vi "UHR-Fleezers Control (host) - 12.0.vi"() -> ()   [LabVIEW 2014] (continued)
                                frame #2 {
                                n432 = property on="Load parameters" class="Bool (strict)"("Val(Sgnl)"=TRUE ("Value (Signaling)")) -> ()  [unwired: 2 in, 2 out]
                                n433 = case shown="True" "Green ON during\nraster?" {
                                frame False {
                                }
                                frame True {
                                n434 = property on="Green ON/Interlacing" class="Bool (strict)"("Val(Sgnl)"=TRUE ("Value (Signaling)")) -> ()  [unwired: 2 in, 2 out]
                                }
                                }
                                }
                                frame #3 {
                                n435 = Wait (ms)(milliseconds to wait=u32 500) -> ()  [unwired: 1 out]
                                }
                                frame #4 {
                                n436 = property on="Trap Raster Scan" class="Bool (strict)"("Val(Sgnl)"=TRUE ("Value (Signaling)")) -> ()  [unwired: 2 in, 2 out]
                                }
                                frame #5 {
                                n437 = Wait (ms)(milliseconds to wait=u32 2000) -> ()  [unwired: 1 out]
                                }
                                frame #6 {
                                n438 = flat-sequence {
                                tunnel: w717 -> [w724]
                                frame #0 {
                                n439 = while {
                                stop <- w720 stop-if-true
                                n440 = local read "Raster Scanning..."() -> (w719:bool)
                                n441 = local read "Saving..."() -> (w722:bool)
                                n442 = Wait (ms)(milliseconds to wait=u32 100) -> ()  [unwired: 1 out]
                                n443 = Not(x=w722) -> (.not. x?=w721:bool)
                                n444 = Not(x=w719) -> (.not. x?=w718:bool)
                                n445 = And(x=w721, y=w718) -> (x .and. y?=w720:bool)
                                }
                                }
                                frame #1 {
                                n446 = local read "Tether"() -> (w725:bool)
                                n447 = case shown="True" w725 {
                                tunnel: w724 -> [_ w727]
                                frame False {
                                n448 = property on="Fish" class="Bool (strict)"("Val(Sgnl)"="Fish again after \nraster break?") -> ()  [unwired: 2 in, 2 out]
                                }
                                frame True {
                                n449 = stacked-sequence {
                                tunnel: w727 -> [_ w731 _ _ _ _ _ _]
                                frame #0 {
                                n450 = property on="Trap D (MHz)" class="DigNum (strict)"("Val(Sgnl)"="Move to D 2 (MHz)") -> ()  [unwired: 2 in, 2 out]
                                n451 = case shown="True" "Flow ON after\ntether testing?" {
                                frame False {
                                }
                                frame True {
                                n452 = property on="Sample Channel\nFlow" class="Bool (strict)"("Val(Sgnl)"=TRUE ("Value (Signaling)")) -> ()  [unwired: 2 in, 2 out]
                                }
                                }
                                }
                                frame #1 {
                                n453 = flat-sequence {
                                tunnel: w731 -> [w732]
                                frame #0 {
                                n454 = case shown="\"6\"" w732 {
                                frame Default {
                                }
                                frame "6" {
                                n455 = flat-sequence {
                                frame #0 {
                                n456 = Wait (ms)(milliseconds to wait=u32 500) -> ()  [unwired: 1 out]
                                }
                                frame #1 {
                                n457 = property on="Green ON/Interlacing" class="Bool (strict)"("Val(Sgnl)"=TRUE ("Green Laser ON/Interlacing")) -> ()  [unwired: 2 in, 2 out]
                                }
                                }
                                }
                                }
                                }
                                frame #1 {
                                n458 = case shown="True" "Save at end (5, 6)" {
                                selector: "Save at end (5, 6)" -> [_ w736]
                                frame False {
                                }
                                frame True {
                                n459 = flat-sequence {
                                tunnel: w736 -> [w738]
                                frame #0 {
                                n460 = Wait (ms)(milliseconds to wait=u32 500) -> ()  [unwired: 1 out]
                                }
                                frame #1 {
                                n461 = local write "Start Saving"(w738) -> ()
                                }
                                }
                                }
                                }
                                }
                                }
                                }
                                frame #2 {
                                n462 = local read "Bead Sep. Int. Time (s)"() -> (w741:dbl)
                                n463 = Multiply(x=w741, y=1000.0) -> (x*y=w740:dbl)
                                n464 = Wait (ms)(milliseconds to wait=w740) -> ()  [unwired: 1 out]
                                }
                                frame #3 {
                                n465 = property on="Remove Offset" class="Bool (strict)"("Val(Sgnl)"=TRUE ("Value (Signaling)")) -> ()  [unwired: 2 in, 2 out]
                                }
                                frame #4 {
                                n466 = property on="Read FX file" class="Bool (strict)"("Val(Sgnl)"=TRUE ("Value (Signaling)")) -> ()  [unwired: 2 in, 2 out]
                                }
                                frame #5 {
                                n467 = Wait (ms)(milliseconds to wait=u32 300) -> ()  [unwired: 1 out]
                                }
                                frame #6 {
                                n468 = local read "Bad fit error"() -> (w750:dbl)
                                n469 = local read "Fit offset"() -> (w753:dbl)
                                n470 = Greater Or Equal?(x=w750, y="Bad fit thresh") -> (x >= y?=→"Bad fit":bool)
                                n471 = Greater Or Equal?(x=w753, y="Fit offset thresh") -> (x >= y?=→"Multiple tether":bool)
                                n472 = local read "Hyst. error"() -> (w747:dbl)
                                n473 = Greater Or Equal?(x=w747, y="Hysteresis thresh") -> (x >= y?=→"Hysteresis":bool)
                                }
                                frame #7 {
                                w758 = 0
                                n474 = local read "Bad fit error"() -> (w760:dbl)
                                n475 = local read "Hyst. error"() -> (w759:dbl)
                                n476 = local read "Fit offset"() -> (w761:dbl)
                                n477 = local read "Multiple tether"() -> (w767:bool)
                                n478 = local read "Hysteresis"() -> (w765:bool)
                                n479 = local read "Bad fit"() -> (w766:bool)
                                n480 = Not(x=w765) -> (.not. x?=w757:bool)
                                n481 = Not(x=w766) -> (.not. x?=w763:bool)
                                n482 = Greater?(x=w761, y=w758) -> (0:w756:bool)
                                n483 = Greater?(x=w760, y=w758) -> (0:w755:bool)
                                n484 = Greater?(x=w759, y=w758) -> (0:w754:bool)
                                n485 = Not(x=w767) -> (.not. x?=w764:bool)
                                n486 = Compound Arithmetic op=AND(w764, w763, w757, w756, w755, w754) -> (w762:bool)
                                "Good tether" <- w762
                                n487 = case shown="True" w762 {
                                frame False {
                                }
                                frame True {
                                n488 = call <vilib>:"Beep.vi"("use system alert? (T)"=FALSE, "duration (msec)"=u32 200, "frequency (Hz)"=u32 2000) -> ()  [unwired: 9 in]
                                }
                                }
                                }
                                }
                                }
                                }
                                }
                                }
                                }
                                }
                                }
                                frame "2", Default {
                                }
                              }
                            }
                            frame #3 {
                              n489 = local read "Multiple tether"() -> (w773:bool)
                              n490 = And(x="Break multiple", y=w773) -> (x .and. y?=w771:bool)
                              n491 = case shown="True" w771 {
                                frame False {
                                }
                                frame True {
                                n492 = stacked-sequence {
                                frame #0 {
                                n493 = property on="Trap D (MHz)" class="DigNum (strict)"("Val(Sgnl)"="Trap D to \nbreak (MHz)") -> ()  [unwired: 2 in, 2 out]
                                }
                                frame #1 {
                                n494 = case shown="True" "Fish after\nmultiple break" {
                                frame False {
                                }
                                frame True {
                                n495 = while {
                                stop <- w778 stop-if-true
                                n496 = local read "Multiple tether"() -> (w780:bool)
                                n497 = local read "Fish"() -> (w777:bool)
                                n498 = local read "Stop All"() -> (w776:bool)
                                n499 = Wait (ms)(milliseconds to wait=u32 100) -> ()  [unwired: 1 out]
                                n500 = Not(x=w780) -> (.not. x?=w779:bool)
                                n501 = Compound Arithmetic op=OR(w776, w779, w777) -> (w778:bool)
                                }
                                }
                                }
                                }
                                frame #2 {
                                n502 = local read "Fish after\nmultiple break"() -> (w785:bool)
                                n503 = local read "Stage Moving"() -> (w784:bool)
                                n504 = Not(x=w784) -> (.not. x?=w782:bool)
                                n505 = And(x=w785, y=w782) -> (x .and. y?=w783:bool)
                                n506 = property on="Fish" class="Bool (strict)"("Val(Sgnl)"=w783) -> ()  [unwired: 2 in, 2 out]
                                }
                                }
                                }
                              }
                            }
                            frame #4 {
                              n507 = local read "Bad fit"() -> (w787:bool)
                              n508 = And(x="Break bad fit", y=w787) -> (x .and. y?=w786:bool)
                              n509 = case shown="True" w786 {
                                frame False {
                                }
                                frame True {
                                n510 = stacked-sequence {
                                frame #0 {
                                n511 = local read "Trap D to \nbreak (MHz)"() -> (w789:dbl)
                                n512 = property on="Trap D (MHz)" class="DigNum (strict)"("Val(Sgnl)"=w789) -> ()  [unwired: 2 in, 2 out]
                                }
                                frame #1 {
                                n513 = case shown="True" "Fish after\nbad fit break?" {
                                frame False {
                                }
                                frame True {
                                n514 = while {
                                stop <- w793 stop-if-true
                                n515 = local read "Stop All"() -> (w791:bool)
                                n516 = local read "Bad fit"() -> (w792:bool)
                                n517 = local read "Fish"() -> (w794:bool)
                                n518 = Not(x=w792) -> (.not. x?=w795:bool)
                                n519 = Wait (ms)(milliseconds to wait=u32 100) -> ()  [unwired: 1 out]
                                n520 = Compound Arithmetic op=OR(w791, w795, w794) -> (w793:bool)
                                }
                                }
                                }
                                }
                                frame #2 {
                                n521 = local read "Fish after\nbad fit break?"() -> (w797:bool)
                                n522 = local read "Stage Moving"() -> (w800:bool)
                                n523 = Not(x=w800) -> (.not. x?=w799:bool)
                                n524 = And(x=w797, y=w799) -> (x .and. y?=w798:bool)
                                n525 = property on="Fish" class="Bool (strict)"("Val(Sgnl)"=w798) -> ()  [unwired: 2 in, 2 out]
                                }
                                }
                                }
                              }
                            }
                            frame #5 {
                              n526 = local read "Hysteresis"() -> (w802:bool)
                              n527 = And(x="Break hyst", y=w802) -> (x .and. y?=w801:bool)
                              n528 = case shown="True" w801 {
                                frame False {
                                }
                                frame True {
                                n529 = stacked-sequence {
                                frame #0 {
                                n530 = local read "Trap D to \nbreak (MHz)"() -> (w804:dbl)
                                n531 = property on="Trap D (MHz)" class="DigNum (strict)"("Val(Sgnl)"=w804) -> ()  [unwired: 2 in, 2 out]
                                }
                                frame #1 {
                                n532 = case shown="True" "Fish ater hyst?" {
                                frame False {
                                }
                                frame True {
                                n533 = while {
                                stop <- w810 stop-if-true
                                n534 = local read "Hysteresis"() -> (w809:bool)
                                n535 = local read "Stop All"() -> (w806:bool)
                                n536 = local read "Fish"() -> (w807:bool)
                                n537 = Wait (ms)(milliseconds to wait=u32 100) -> ()  [unwired: 1 out]
                                n538 = Not(x=w809) -> (.not. x?=w808:bool)
                                n539 = Compound Arithmetic op=OR(w806, w808, w807) -> (w810:bool)
                                }
                                }
                                }
                                }
                                frame #2 {
                                n540 = local read "Fish ater hyst?"() -> (w815:bool)
                                n541 = local read "Stage Moving"() -> (w814:bool)
                                n542 = Not(x=w814) -> (.not. x?=w813:bool)
                                n543 = And(x=w815, y=w813) -> (x .and. y?=w812:bool)
                                n544 = property on="Fish" class="Bool (strict)"("Val(Sgnl)"=w812) -> ()  [unwired: 2 in, 2 out]
                                }
                                }
                                }
                              }
                            }
                            frame #6 {
                              n545 = local read "Good tether"() -> (w816:bool)
                              n546 = case shown="True" w816 {
                                frame False {
                                }
                                frame True {
                                n547 = case shown="\"1\"" "If good, then:" {
                                frame "0", Default {
                                }
                                frame "1" {
                                n548 = property on="Force FB Script" class="Bool (strict)"("Val(Sgnl)"=TRUE ("Value (Signaling)")) -> ()  [unwired: 2 in, 2 out]
                                }
                                }
                                }
                              }
                            }
                          }
                        }
                        frame "7" {
                          n549 = property on="Force FB Script" class="Bool (strict)"("Val(Sgnl)"=TRUE ("Value (Signaling)")) -> ()  [unwired: 2 in, 2 out]
                        }
                        frame "8" {
                          n550 = property on="Fixed Traps Script" class="Bool (strict)"("Val(Sgnl)"=TRUE ("Value (Signaling)")) -> ()  [unwired: 2 in, 2 out]
                        }
                      }
                      "Tether" <- "Tether Alarm?"
                    }
                  }
                }
                frame #2 {
                  n551 = local read "Oscillate Set 1"() -> (w826:bool)
                  n552 = local read "Stop All"() -> (w824:bool)
                  n553 = Or(x=w826, y=w821) -> (x .or. y?=w823:bool)
                  n554 = Not(x=w823) -> (.not. x?=w825:bool)
                  n555 = Compound Arithmetic op=OR(w824, w825) -> (w822:bool)
                }
              }
              n556 = node-c288() -> ()  [unwired: 2 out]
            }
            n557 = node-c288(w576) -> ()  [unwired: 1 out]
          }
        }
      }
      event "Fl. Triggered...": Value Change {
        n558 = event-data() -> ()  [unwired: 7 out]
        n559 = case shown="True" "Fl. Triggered..." {
          frame False {
          }
          frame True {
            n560 = node-c288() -> (w837:T26)  [unwired: 4 out]
            n561 = timed-loop {
              timing: w837 -> [_]
              timing-out: [_] -> w836
              tunnel: "Action" -> [w845]
              shift-right: [w842] -> _
              shift-left: u8 255 -> [w844]
              shift-right: [w839] -> _
              shift-left: 255 -> [w841]
              stop <- w838 stop-if-true
              # "Reset confocal spot"
              n562 = node-c288() -> ()  [unwired: 2 out]
              n563 = flat-sequence {
                tunnel: w845 -> [w865]
                tunnel: w844 -> [w864]
                tunnel: [w863] -> w843
                tunnel: w841 -> [w850]
                tunnel: [w849] -> w840
                tunnel: [w1249] -> w838
                tunnel: w843 -> [w1248]
                tunnel: [w1248] -> w842
                tunnel: [w1247] -> w839
                tunnel: w840 -> [w1247]
                frame #0 {
                  n564 = local read "Delta Fl. 2"() -> (w862:dbl)
                  n565 = local read "Delta Fl. 1"() -> (w857:dbl)
                  n566 = Multiply(x="Fl. D Thresh. (kHz)", y=1000.0) -> (x*y=w852:dbl)
                  n567 = Select(t=w857, s="APD to Watch", f=w862) -> (s? t:f=w853:dbl)
                  n568 = Greater?(x=w853, y=w852) -> (0:w858:bool)
                  n569 = Or(x="Force Yank", y=w858) -> (x .or. y?=w856:bool)
                  n570 = And(x=w856, y="Yank when?") -> (x .and. y?=w854:bool)
                  n571 = case shown="False" w854 {
                    tunnel: w865 -> [w868 w1071]
                    tunnel: w864 -> [w870 w1067]
                    tunnel: [w870 w1065] -> w863
                    tunnel: w853 -> [w876 _]
                    tunnel: w852 -> [w875 _]
                    tunnel: "Force Yank" -> [w873 _]
                    tunnel: w850 -> [w872 w1064]
                    tunnel: [w871 w1064] -> w849
                    frame False {
                      n572 = Negate(x=w875) -> (-x=w867:dbl)
                      n573 = local write "Fl. High"(TRUE ("Fl. High")) -> ()
                      n574 = Less?(x=w876, y=w867) -> (x < y?=w874:bool)
                      n575 = Or(x=w873, y=w874) -> (x .or. y?=w869:bool)
                      n576 = case shown="True" w869 {
                        tunnel: w872 -> [w877 w887]
                        tunnel: [w877 w886] -> w871
                        tunnel: w868 -> [_ w885]
                        frame False {
                        }
                        frame True {
                          n577 = flat-sequence {
                            tunnel: w887 -> [w893]
                            tunnel: w885 -> [w890]
                            tunnel: [w892] -> w884
                            tunnel: [w891] -> w883
                            tunnel: [w890] -> w882
                            tunnel: w881 -> [w889]
                            tunnel: [w889] -> w880
                            tunnel: w879 -> [w888]
                            tunnel: [w888] -> w878
                            tunnel: [w965] -> w886
                            tunnel: w884 -> [w965]
                            tunnel: w883 -> [w964]
                            tunnel: w882 -> [w963]
                            tunnel: w880 -> [w962]
                            tunnel: w878 -> [w961]
                            frame #0 {
                              n578 = call <vilib>:"Beep.vi"() -> ()  [unwired: 12 in]
                              n579 = local write "Waiting"(FALSE ("Waiting")) -> ()
                              n580 = Increment(x=w893) -> (x+1=w892:i32)
                              n581 = case shown="\"Yank\"" w890 {
                                tunnel: w892 -> [_ w898 _]
                                frame "Alarm", Default {
                                }
                                frame "Yank" {
                                n582 = flat-sequence {
                                tunnel: w898 -> [w901]
                                tunnel: [w900] -> w897
                                tunnel: [w899] -> w896
                                tunnel: w897 -> [w911]
                                tunnel: w896 -> [w912]
                                frame #0 {
                                n583 = local read "Yank Delay (s)"() -> (w904:dbl)
                                n584 = local read "N Array El"() -> (w899:u8)
                                n585 = Quotient & Remainder(x=w901, y=w899) -> (x-y*floor(x/y)=w900:i32)  [unwired: 1 out]
                                n586 = Multiply(x=w904, y=1000.0) -> (x*y=w902:dbl)
                                n587 = Wait (ms)(milliseconds to wait=w902) -> ()  [unwired: 1 out]
                                }
                                frame #1 {
                                n588 = local read "Yank to which?"() -> (w906:bool)
                                n589 = local read "Random Choice"() -> (w916:bool)
                                n590 = local read "Yank to Trap D (MHz)"() -> (w909:dbl[])
                                n591 = local read "Yank to SP"() -> (w910:dbl[])
                                n592 = Random Number (0-1)() -> (number: 0 to 1=w915:dbl)
                                n593 = Multiply(x=w912, y=w915) -> (x*y=w914:dbl)
                                n594 = Round Toward -Infinity(1:w914) -> (0:w913:dbl)
                                n595 = Select(t=w913, s=w916, f=w911) -> (s? t:f=w907:dbl)
                                n596 = Select(t=w909, s=w906, f=w910) -> (s? t:f=w908:dbl[])
                                n597 = Index Array(array=w908, index=w907) -> (element=w905:dbl)
                                n598 = case shown="False" w906 {
                                tunnel: w905 -> [w917 w945]
                                frame False {
                                n599 = flat-sequence {
                                tunnel: w917 -> [w918]
                                frame #0 {
                                n600 = property on="Trap Pos FB SP" class="DigNum (strict)"("Val(Sgnl)"=w918) -> ()  [unwired: 2 in, 2 out]
                                }
                                frame #1 {
                                n601 = Wait (ms)(milliseconds to wait=u32 700) -> ()  [unwired: 1 out]
                                }
                                frame #2 {
                                n602 = local read "Action (%)"() -> (w923:dbl)
                                n603 = Absolute Value(x=w923) -> (abs(x)=w922:dbl)
                                n604 = Greater?(x=w922, y=70.0) -> (0:w920:bool)
                                n605 = property on="Remove Action Offset" class="Bool (strict)"("Val(Sgnl)"=w920) -> ()  [unwired: 2 in, 2 out]
                                }
                                frame #3 {
                                n606 = for {
                                N: 4 -> [_]
                                n607 = flat-sequence {
                                frame #0 {
                                n608 = Wait (ms)(milliseconds to wait=u32 500) -> ()  [unwired: 1 out]
                                }
                                frame #1 {
                                n609 = local read "Action (%)"() -> (w929:dbl)
                                n610 = Absolute Value(x=w929) -> (abs(x)=w928:dbl)
                                n611 = Greater?(x=w928, y=70.0) -> (0:w926:bool)
                                n612 = property on="Remove Action Offset" class="Bool (strict)"("Val(Sgnl)"=w926) -> ()  [unwired: 2 in, 2 out]
                                }
                                }
                                }
                                }
                                frame #4 {
                                n613 = Wait (ms)(milliseconds to wait=u32 500) -> ()  [unwired: 1 out]
                                }
                                frame #5 {
                                n614 = local read "Mean"() -> (w937:dbl)
                                n615 = Greater?(x=w937, y=11.0) -> (0:w931:bool)
                                n616 = Not(x=w931) -> (.not. x?=w932:bool)
                                n617 = And(x=w932, y="Shift confocal") -> (x .and. y?=w934:bool)
                                n618 = And(x=w931, y="Shift confocal") -> (x .and. y?=w935:bool)
                                n619 = case shown="True" w935 {
                                frame False {
                                }
                                frame True {
                                n620 = local read "Confocal Y 2 (V)"() -> (w941:dbl)
                                n621 = local read "Confocal X 2 (V)"() -> (w940:dbl)
                                n622 = property on="AO1" class="Slide (strict)"("Val(Sgnl)"=w941) -> ()  [unwired: 2 in, 2 out]
                                n623 = property on="AO2" class="Slide (strict)"("Val(Sgnl)"=w940) -> ()  [unwired: 2 in, 2 out]
                                }
                                }
                                n624 = case shown="True" w934 {
                                frame False {
                                }
                                frame True {
                                n625 = local read "Confocal Y 1 (V)"() -> (w939:dbl)
                                n626 = local read "Confocal X 1 (V)"() -> (w938:dbl)
                                n627 = property on="AO1" class="Slide (strict)"("Val(Sgnl)"=w939) -> ()  [unwired: 2 in, 2 out]
                                n628 = property on="AO2" class="Slide (strict)"("Val(Sgnl)"=w938) -> ()  [unwired: 2 in, 2 out]
                                }
                                }
                                }
                                frame #6 {
                                n629 = Wait (ms)(milliseconds to wait=u32 1500) -> ()  [unwired: 1 out]
                                }
                                frame #7 {
                                n630 = property on="Rem fb disp offset" class="Bool (strict)"("Val(Sgnl)"=TRUE ("Value (Signaling)")) -> ()  [unwired: 2 in, 2 out]
                                n631 = property on="Remove Offset" class="Bool (strict)"("Val(Sgnl)"=TRUE ("Value (Signaling)")) -> ()  [unwired: 2 in, 2 out]
                                }
                                }
                                }
                                frame True {
                                n632 = flat-sequence {
                                tunnel: w945 -> [w946]
                                frame #0 {
                                n633 = property on="Trap D (MHz)" class="DigNum (strict)"("Val(Sgnl)"=w946) -> ()  [unwired: 2 in, 2 out]
                                }
                                frame #1 {
                                n634 = Wait (ms)(milliseconds to wait=u32 500) -> ()  [unwired: 1 out]
                                }
                                frame #2 {
                                n635 = local read "Shift confocal"() -> (w952:bool)
                                n636 = local read "Mean"() -> (w954:dbl)
                                n637 = Greater?(x=w954, y=11.0) -> (0:w951:bool)
                                n638 = Not(x=w951) -> (.not. x?=w950:bool)
                                n639 = And(x=w950, y=w952) -> (x .and. y?=w948:bool)
                                n640 = And(x=w951, y=w952) -> (x .and. y?=w949:bool)
                                n641 = case shown="True" w949 {
                                frame False {
                                }
                                frame True {
                                n642 = local read "Confocal Y 2 (V)"() -> (w958:dbl)
                                n643 = local read "Confocal X 2 (V)"() -> (w957:dbl)
                                n644 = property on="AO2" class="Slide (strict)"("Val(Sgnl)"=w957) -> ()  [unwired: 2 in, 2 out]
                                n645 = property on="AO1" class="Slide (strict)"("Val(Sgnl)"=w958) -> ()  [unwired: 2 in, 2 out]
                                }
                                }
                                n646 = case shown="True" w948 {
                                frame False {
                                }
                                frame True {
                                n647 = local read "Confocal X 1 (V)"() -> (w955:dbl)
                                n648 = local read "Confocal Y 1 (V)"() -> (w956:dbl)
                                n649 = property on="AO2" class="Slide (strict)"("Val(Sgnl)"=w955) -> ()  [unwired: 2 in, 2 out]
                                n650 = property on="AO1" class="Slide (strict)"("Val(Sgnl)"=w956) -> ()  [unwired: 2 in, 2 out]
                                }
                                }
                                }
                                }
                                }
                                }
                                }
                                }
                                }
                                frame "Image" {
                                n651 = property on="Confocal\nImage" class="Bool (strict)"("Val(Sgnl)"=TRUE ("Value (Signaling)")) -> ()  [unwired: 2 in, 2 out]
                                }
                              }
                              n652 = local write "Fl. High"(FALSE ("Fl. High")) -> ()
                              n653 = local read "Time (s)"() -> (w891:dbl)
                            }
                            frame #1 {
                              n654 = case shown="True" "Auto F Reset" {
                                tunnel: w964 -> [_ w969]
                                tunnel: w963 -> [_ w968]
                                tunnel: w962 -> [_ w967]
                                tunnel: w961 -> [_ w966]
                                frame False {
                                }
                                frame True {
                                n655 = node-c288() -> (w971:T26)  [unwired: 4 in]
                                n656 = timed-loop {
                                timing: w971 -> [_]
                                timing-out: [_] -> w970
                                tunnel: w969 -> [w976]
                                tunnel: w968 -> [w975]
                                tunnel: w967 -> [w974]
                                tunnel: w966 -> [w973]
                                stop <- w972 stop-if-true
                                n657 = node-c288() -> ()  [unwired: 1 in, 1 out]
                                n658 = local read "APD to Watch"() -> (w986:bool)
                                n659 = local read "Fl. D Thresh. (kHz)"() -> (w985:dbl)
                                n660 = local read "Delta Fl. 1"() -> (w987:dbl)
                                n661 = local read "Delta Fl. 2"() -> (w988:dbl)
                                n662 = local read "Fl. Triggered..."() -> (w979:bool)
                                n663 = local read "Stop All"() -> (w980:bool)
                                n664 = local read "Reset Force"() -> (w978:bool)
                                n665 = Multiply(x=w985, y=1000.0) -> (x*y=w983:dbl)
                                n666 = Not(x=w979) -> (.not. x?=w977:bool)
                                n667 = Select(t=w987, s=w986, f=w988) -> (s? t:f=w982:dbl)
                                n668 = Greater?(x=w982, y=w983) -> (0:w981:bool)
                                n669 = Compound Arithmetic op=OR(w981, w980, w977, w978) -> (w972:bool)
                                n670 = case shown="True" w972 {
                                tunnel: w976 -> [_ w992]
                                tunnel: w975 -> [_ w996]
                                tunnel: w974 -> [_ w995]
                                tunnel: w973 -> [_ w994]
                                frame False {
                                }
                                frame True {
                                n671 = case shown="\"Yank\"" w996 {
                                tunnel: w995 -> [_ w1006]
                                tunnel: w994 -> [_ w1004]
                                frame "Image", Default {
                                }
                                frame "Yank" {
                                n672 = flat-sequence {
                                tunnel: [w1009] -> w1007
                                tunnel: w1006 -> [w1009]
                                tunnel: [w1008] -> w1005
                                tunnel: w1004 -> [w1008]
                                tunnel: w1007 -> [w1015]
                                tunnel: w1005 -> [w1013]
                                frame #0 {
                                n673 = local read "Yank Delay (s)"() -> (w1012:dbl)
                                n674 = Multiply(x=w1012, y=1000.0) -> (x*y=w1010:dbl)
                                n675 = Wait (ms)(milliseconds to wait=w1010) -> ()  [unwired: 1 out]
                                }
                                frame #1 {
                                n676 = local read "Yank to which?"() -> (w1014:bool)
                                n677 = case shown="False" w1014 {
                                tunnel: w1015 -> [_ w1044]
                                tunnel: w1013 -> [w1016 _]
                                frame False {
                                n678 = flat-sequence {
                                tunnel: w1016 -> [w1017]
                                frame #0 {
                                n679 = property on="Trap Pos FB SP" class="DigNum (strict)"("Val(Sgnl)"=w1017) -> ()  [unwired: 2 in, 2 out]
                                }
                                frame #1 {
                                n680 = Wait (ms)(milliseconds to wait=u32 700) -> ()  [unwired: 1 out]
                                }
                                frame #2 {
                                n681 = local read "Action (%)"() -> (w1022:dbl)
                                n682 = Absolute Value(x=w1022) -> (abs(x)=w1021:dbl)
                                n683 = Greater?(x=w1021, y=70.0) -> (0:w1019:bool)
                                n684 = property on="Remove Action Offset" class="Bool (strict)"("Val(Sgnl)"=w1019) -> ()  [unwired: 2 in, 2 out]
                                }
                                frame #3 {
                                n685 = for {
                                N: 4 -> [_]
                                n686 = flat-sequence {
                                frame #0 {
                                n687 = Wait (ms)(milliseconds to wait=u32 500) -> ()  [unwired: 1 out]
                                }
                                frame #1 {
                                n688 = local read "Action (%)"() -> (w1028:dbl)
                                n689 = Absolute Value(x=w1028) -> (abs(x)=w1027:dbl)
                                n690 = Greater?(x=w1027, y=70.0) -> (0:w1025:bool)
                                n691 = property on="Remove Action Offset" class="Bool (strict)"("Val(Sgnl)"=w1025) -> ()  [unwired: 2 in, 2 out]
                                }
                                }
                                }
                                }
                                frame #4 {
                                n692 = Wait (ms)(milliseconds to wait=u32 500) -> ()  [unwired: 1 out]
                                }
                                frame #5 {
                                n693 = local read "Shift confocal"() -> (w1033:bool)
                                n694 = local read "Mean"() -> (w1036:dbl)
                                n695 = Greater?(x=w1036, y=11.0) -> (0:w1032:bool)
                                n696 = Not(x=w1032) -> (.not. x?=w1031:bool)
                                n697 = And(x=w1032, y=w1033) -> (x .and. y?=w1034:bool)
                                n698 = And(x=w1031, y=w1033) -> (x .and. y?=w1030:bool)
                                n699 = case shown="True" w1034 {
                                frame False {
                                }
                                frame True {
                                n700 = local read "Confocal X 2 (V)"() -> (w1039:dbl)
                                n701 = local read "Confocal Y 2 (V)"() -> (w1040:dbl)
                                n702 = property on="AO2" class="Slide (strict)"("Val(Sgnl)"=w1039) -> ()  [unwired: 2 in, 2 out]
                                n703 = property on="AO1" class="Slide (strict)"("Val(Sgnl)"=w1040) -> ()  [unwired: 2 in, 2 out]
                                }
                                }
                                n704 = case shown="True" w1030 {
                                frame False {
                                }
                                frame True {
                                n705 = local read "Confocal Y 1 (V)"() -> (w1038:dbl)
                                n706 = local read "Confocal X 1 (V)"() -> (w1037:dbl)
                                n707 = property on="AO1" class="Slide (strict)"("Val(Sgnl)"=w1038) -> ()  [unwired: 2 in, 2 out]
                                n708 = property on="AO2" class="Slide (strict)"("Val(Sgnl)"=w1037) -> ()  [unwired: 2 in, 2 out]
                                }
                                }
                                }
                                frame #6 {
                                n709 = Wait (ms)(milliseconds to wait=u32 1500) -> ()  [unwired: 1 out]
                                }
                                frame #7 {
                                n710 = property on="Remove Offset" class="Bool (strict)"("Val(Sgnl)"=TRUE ("Value (Signaling)")) -> ()  [unwired: 2 in, 2 out]
                                n711 = property on="Rem fb disp offset" class="Bool (strict)"("Val(Sgnl)"=TRUE ("Value (Signaling)")) -> ()  [unwired: 2 in, 2 out]
                                }
                                }
                                }
                                frame True {
                                n712 = flat-sequence {
                                tunnel: w1044 -> [w1045]
                                frame #0 {
                                n713 = property on="Trap D (MHz)" class="DigNum (strict)"("Val(Sgnl)"=w1045) -> ()  [unwired: 2 in, 2 out]
                                }
                                frame #1 {
                                n714 = Wait (ms)(milliseconds to wait=u32 500) -> ()  [unwired: 1 out]
                                }
                                frame #2 {
                                n715 = local read "Shift confocal"() -> (w1051:bool)
                                n716 = local read "Mean"() -> (w1052:dbl)
                                n717 = Greater?(x=w1052, y=11.0) -> (0:w1050:bool)
                                n718 = And(x=w1050, y=w1051) -> (x .and. y?=w1048:bool)
                                n719 = Not(x=w1050) -> (.not. x?=w1049:bool)
                                n720 = And(x=w1049, y=w1051) -> (x .and. y?=w1047:bool)
                                n721 = case shown="True" w1048 {
                                frame False {
                                }
                                frame True {
                                n722 = local read "Confocal Y 2 (V)"() -> (w1057:dbl)
                                n723 = local read "Confocal X 2 (V)"() -> (w1056:dbl)
                                n724 = property on="AO1" class="Slide (strict)"("Val(Sgnl)"=w1057) -> ()  [unwired: 2 in, 2 out]
                                n725 = property on="AO2" class="Slide (strict)"("Val(Sgnl)"=w1056) -> ()  [unwired: 2 in, 2 out]
                                }
                                }
                                n726 = case shown="True" w1047 {
                                frame False {
                                }
                                frame True {
                                n727 = local read "Confocal Y 1 (V)"() -> (w1055:dbl)
                                n728 = local read "Confocal X 1 (V)"() -> (w1054:dbl)
                                n729 = property on="AO2" class="Slide (strict)"("Val(Sgnl)"=w1054) -> ()  [unwired: 2 in, 2 out]
                                n730 = property on="AO1" class="Slide (strict)"("Val(Sgnl)"=w1055) -> ()  [unwired: 2 in, 2 out]
                                }
                                }
                                }
                                }
                                }
                                }
                                }
                                }
                                }
                                }
                                n731 = local read "Time (s)"() -> (w991:dbl)
                                n732 = Subtract(x=w992, y=w991) -> (x-y=w1003:dbl)
                                n733 = Number To Decimal String(number=w1003, width (-)=i16 0) -> (decimal integer string=w1001:string)
                                n734 = Concatenate Strings(w1001, " s fluorescence event") -> (w998:string)
                                n735 = local read "Messages"() -> (w999:string)
                                n736 = local write "Duration (s)"(w1003) -> ()
                                n737 = call "Update messages.vi"("Message to add"=w998, "Old message string"=w999) -> ("New message string"=w997:string)
                                n738 = local write "Messages"(w997) -> ()
                                n739 = call <vilib>:"Beep.vi"() -> ()  [unwired: 12 in]
                                n740 = local write "Reset Force"(FALSE ("Force Reset")) -> ()
                                n741 = local write "Fl. High"(TRUE ("Fl. High")) -> ()
                                n742 = local write "Waiting"(TRUE ("Waiting")) -> ()
                                }
                                }
                                n743 = node-c288() -> ()  [unwired: 1 in, 1 out]
                                }
                                n744 = node-c288(w970) -> ()  [unwired: 1 out]
                                }
                              }
                            }
                          }
                          n745 = local read "Trap Pos FB SP"() -> (w879:fxp<+/-,16,1>)
                          n746 = local read "Trap D (MHz)"() -> (w881:dbl)
                        }
                      }
                    }
                    frame True {
                      n747 = flat-sequence {
                        tunnel: w1068 -> [w1078]
                        tunnel: [w1078] -> w1072
                        tunnel: w1071 -> [w1077]
                        tunnel: [w1077] -> w1070
                        tunnel: [w1076] -> w1069
                        tunnel: w1067 -> [w1075]
                        tunnel: [w1074] -> w1066
                        tunnel: w1063 -> [w1073]
                        tunnel: [w1073] -> w1062
                        tunnel: w1072 -> [w1150]
                        tunnel: w1070 -> [w1149]
                        tunnel: w1069 -> [w1148]
                        tunnel: w1066 -> [w1147]
                        tunnel: w1062 -> [w1146]
                        tunnel: [w1147] -> w1065
                        frame #0 {
                          n748 = call <vilib>:"Beep.vi"() -> ()  [unwired: 3 in, 9 out]
                          n749 = local write "Waiting"(FALSE ("Waiting")) -> ()
                          n750 = Increment(x=w1075) -> (x+1=w1074:u8)
                          n751 = case shown="\"Image\"" w1077 {
                            tunnel: w1074 -> [_ _ w1084 _]
                            frame "Image" {
                              n752 = property on="Confocal\nImage" class="Bool (strict)"("Val(Sgnl)"=TRUE ("Value (Signaling)")) -> ()  [unwired: 2 in, 2 out]
                            }
                            frame "Alarm", Default {
                            }
                            frame "Yank" {
                              n753 = flat-sequence {
                                tunnel: w1084 -> [w1087]
                                tunnel: [w1086] -> w1083
                                tunnel: ["N Array El"] -> w1082
                                tunnel: w1083 -> [w1101]
                                tunnel: w1082 -> [w1097]
                                frame #0 {
                                n754 = Multiply(x="Yank Delay (s)", y=1000.0) -> (x*y=w1090:dbl)
                                n755 = Quotient & Remainder(x=w1087, y="N Array El") -> (x-y*floor(x/y)=w1086:u8)  [unwired: 1 out]
                                n756 = Wait (ms)(milliseconds to wait=w1090) -> ()  [unwired: 1 out]
                                }
                                frame #1 {
                                n757 = Random Number (0-1)() -> (number: 0 to 1=w1098:dbl)
                                n758 = Multiply(x=w1097, y=w1098) -> (x*y=w1096:dbl)
                                n759 = Round Toward -Infinity(1:w1096) -> (0:w1095:dbl)
                                n760 = Select(t=w1095, s="Random Choice", f=w1101) -> (s? t:f=w1099:dbl)
                                n761 = Select(t="Yank to Trap D (MHz)", s="Yank to which?", f="Yank to SP") -> (s? t:f=w1092:dbl[])
                                n762 = Index Array(array=w1092, index=w1099) -> (element=w1102:dbl)
                                n763 = case shown="False" "Yank to which?" {
                                tunnel: w1102 -> [w1103 w1130]
                                frame False {
                                n764 = flat-sequence {
                                tunnel: w1103 -> [w1104]
                                frame #0 {
                                n765 = property on="Trap Pos FB SP" class="DigNum (strict)"("Val(Sgnl)"=w1104) -> ()  [unwired: 2 in, 2 out]
                                }
                                frame #1 {
                                n766 = Wait (ms)(milliseconds to wait=u32 700) -> ()  [unwired: 1 out]
                                }
                                frame #2 {
                                n767 = local read "Action (%)"() -> (w1109:dbl)
                                n768 = Absolute Value(x=w1109) -> (abs(x)=w1108:dbl)
                                n769 = Greater?(x=w1108, y=70.0) -> (0:w1106:bool)
                                n770 = property on="Remove Action Offset" class="Bool (strict)"("Val(Sgnl)"=w1106) -> ()  [unwired: 2 in, 2 out]
                                }
                                frame #3 {
                                n771 = for {
                                N: 4 -> [_]
                                n772 = flat-sequence {
                                frame #0 {
                                n773 = Wait (ms)(milliseconds to wait=u32 500) -> ()  [unwired: 1 out]
                                }
                                frame #1 {
                                n774 = local read "Action (%)"() -> (w1115:dbl)
                                n775 = Absolute Value(x=w1115) -> (abs(x)=w1114:dbl)
                                n776 = Greater?(x=w1114, y=70.0) -> (0:w1112:bool)
                                n777 = property on="Remove Action Offset" class="Bool (strict)"("Val(Sgnl)"=w1112) -> ()  [unwired: 2 in, 2 out]
                                }
                                }
                                }
                                }
                                frame #4 {
                                n778 = local read "Shift confocal"() -> (w1119:bool)
                                n779 = local read "Mean"() -> (w1122:dbl)
                                n780 = Greater?(x=w1122, y=11.0) -> (0:w1118:bool)
                                n781 = Not(x=w1118) -> (.not. x?=w1117:bool)
                                n782 = And(x=w1117, y=w1119) -> (x .and. y?=w1116:bool)
                                n783 = And(x=w1118, y=w1119) -> (x .and. y?=w1120:bool)
                                n784 = case shown="True" w1120 {
                                frame False {
                                }
                                frame True {
                                n785 = local read "Confocal X 2 (V)"() -> (w1125:dbl)
                                n786 = local read "Confocal Y 2 (V)"() -> (w1126:dbl)
                                n787 = property on="AO2" class="Slide (strict)"("Val(Sgnl)"=w1125) -> ()  [unwired: 2 in, 2 out]
                                n788 = property on="AO1" class="Slide (strict)"("Val(Sgnl)"=w1126) -> ()  [unwired: 2 in, 2 out]
                                }
                                }
                                n789 = case shown="True" w1116 {
                                frame False {
                                }
                                frame True {
                                n790 = local read "Confocal X 1 (V)"() -> (w1123:dbl)
                                n791 = local read "Confocal Y 1 (V)"() -> (w1124:dbl)
                                n792 = property on="AO1" class="Slide (strict)"("Val(Sgnl)"=w1124) -> ()  [unwired: 2 in, 2 out]
                                n793 = property on="AO2" class="Slide (strict)"("Val(Sgnl)"=w1123) -> ()  [unwired: 2 in, 2 out]
                                }
                                }
                                }
                                frame #5 {
                                n794 = Wait (ms)(milliseconds to wait=u32 1500) -> ()  [unwired: 1 out]
                                }
                                frame #6 {
                                n795 = property on="Remove Offset" class="Bool (strict)"("Val(Sgnl)"=TRUE ("Value (Signaling)")) -> ()  [unwired: 2 in, 2 out]
                                n796 = property on="Rem fb disp offset" class="Bool (strict)"("Val(Sgnl)"=TRUE ("Value (Signaling)")) -> ()  [unwired: 2 in, 2 out]
                                }
                                }
                                }
                                frame True {
                                n797 = flat-sequence {
                                tunnel: w1130 -> [w1131]
                                frame #0 {
                                n798 = property on="Trap D (MHz)" class="DigNum (strict)"("Val(Sgnl)"=w1131) -> ()  [unwired: 2 in, 2 out]
                                }
                                frame #1 {
                                n799 = Wait (ms)(milliseconds to wait=u32 500) -> ()  [unwired: 1 out]
                                }
                                frame #2 {
                                n800 = local read "Shift confocal"() -> (w1135:bool)
                                n801 = local read "Mean"() -> (w1133:dbl)
                                n802 = Greater?(x=w1133, y=11.0) -> (0:w1136:bool)
                                n803 = Not(x=w1136) -> (.not. x?=w1137:bool)
                                n804 = And(x=w1137, y=w1135) -> (x .and. y?=w1139:bool)